vi "Core_Chem_User_Interface_v1.4.vi"() -> ()   [LabVIEW 2014] (continued)
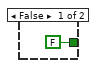
[diagram p11: hidden frame]
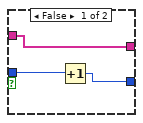
[diagram p16: hidden frame]
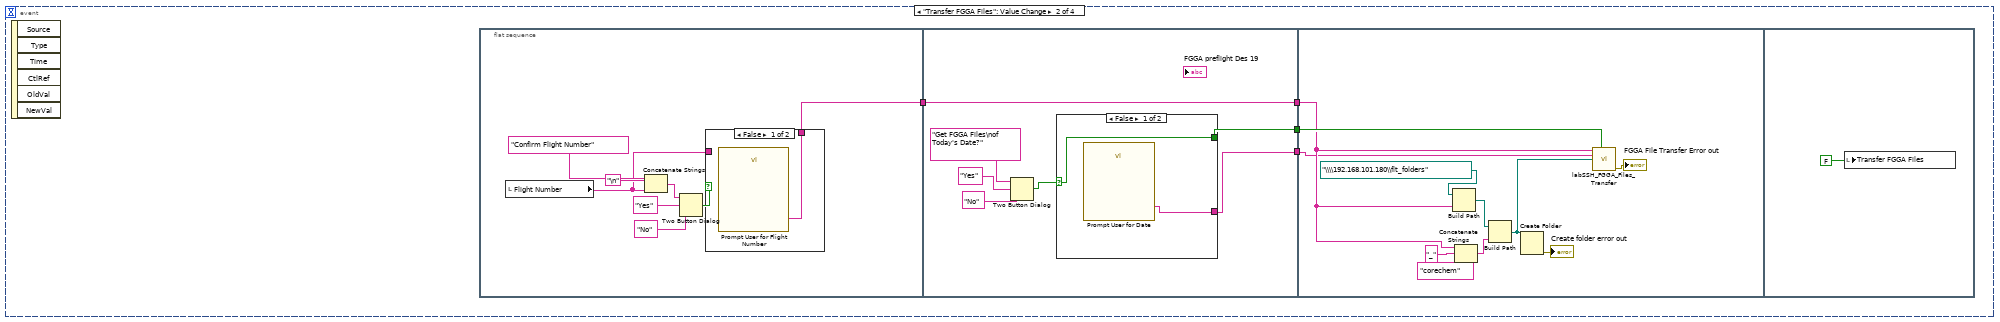
[diagram p18: hidden frame]
            n532 = for {
              N: 60 -> [w1367]
              i -> [w1366]
              n533 = Subtract(x=w1367, y=w1366) -> (x-y=w1365:i32)
              n534 = Decrement(x=w1365) -> (x-1=→"Target Cal\nCal Time Remain (sec)":i32)
              n535 = Wait (ms)(milliseconds to wait=u32 1000) -> ()  [unwired: 1 out]
            }
          }
          frame #5 {
            w1375 = FALSE
            n536 = Cluster To Array(cluster=cluster{"Message 3":string, "Message":string} {"Message 3"="V4", "Message"="V1"}) -> (array=w1373:string[])
            n537 = for {
              tunnel: w1373 -> [w1381] mode=indexing
              tunnel: [w1380] -> w1369
              tunnel: [w1379] -> w1370
              tunnel: w1375 -> [w1378]
              tunnel: w1372 -> [w1377]
              tunnel: w1371 -> [w1376]
              n538 = Bundle(cluster=T4 {"Message"="", "Message Data"=variant} ("Message Cluster"), "Message"=w1381, "Message Data"=w1378) -> (w1383:T4)
              n539 = Enqueue Element(queue=w1377, element=w1383, error in (no error)=w1376) -> (queue out=w1380:refnum<queue>, error out=w1379:errorcluster)  [unwired: 1 in, 1 out]
            }
            n540 = local write "eV4"(w1375) -> ()
            n541 = local write "eV1"(w1375) -> ()
          }
          frame #6 {
            w1385 = 0.0 ("MFC_1\nSLPM Value")
            n542 = local write "MFC_1\nSLPM Value"(w1385) -> ()
            n543 = Bundle(cluster=T4 {"Message"="", "Message Data"=variant} ("Message Cluster"), "Message"="MFC_1", "Message Data"=w1385) -> (w1389:T4)
            n544 = Enqueue Element(queue=w1387, element=w1389, error in (no error)=w1386) -> (error out=w1384:errorcluster)  [unwired: 1 in, 2 out]
          }
          frame #7 {
            n545 = local write "Target Cal"(FALSE ("High Cal")) -> ()
          }
        }
      }
      event "MFC_1\nSLPM Value": Value Change {
        n546 = event-data() -> ()  [unwired: 1 in, 1 out]
        n547 = local read "MFC_1\nSLPM Value"() -> (w1393:dbl)
        n548 = Bundle(cluster=T4 {"Message"="", "Message Data"=variant} ("Message Cluster"), "Message"="MFC_1", "Message Data"=w1393) -> (w1397:T4)
        n549 = Enqueue Element(queue=w1396, element=w1397, error in (no error)=w1395) -> (error out=w1394:errorcluster)  [unwired: 1 in, 2 out]
      }
      event "FGGA UDP Time Offset": Value Change {
        n550 = event-data() -> ("NewVal"=w1400:i32)  [unwired: 1 in, 5 out]
        n551 = Bundle(cluster=T4 {"Message"="", "Message Data"=variant} ("Message Cluster"), "Message"="UDP Time Offset", "Message Data"=w1400) -> (w1404:T4)
        n552 = Enqueue Element(queue=w1403, element=w1404, error in (no error)=w1402) -> (error out=w1401:errorcluster)  [unwired: 1 in, 2 out]
      }
    }
    "FGGA Event Error out" <- w687
  }
  n553 = Create Network Stream Writer Endpoint(6:w53, 7:10 ("writer buffer size"), 9:w55, 10:"//192.168.101.17/command/reader/FGGA" ("reader url"), 11:"/command/writer/FGGA" ("writer name")) -> (0:w52:errorcluster, 3:w51:refnum<k21>)  [unwired: 2 in]
  n554 = node-c288(w11) -> ()  [unwired: 1 out]
  n555 = while {
    tunnel: w2 -> [w1414]
    shift-right: [w1409] -> _
    shift-left: w51 -> [w1411]
    shift-right: [w1407] -> w48
    shift-left: w52 -> [w1413]
    tunnel: w1 -> [w1408]
    stop <- w1407 stop-if-true
    # "FGGA UI Command Sender"
    n556 = Dequeue Element(queue=w1414, error in (no error)=w1408) -> (element=w1410:T4)  [unwired: 1 in, 3 out]
    n557 = Unbundle By Name(w1410) -> ("Message"=w1412:string)
    n558 = case shown="\"UDP Time Offset\"" w1412 {
      tunnel: w1413 -> [w1415 w1419 w1426 w1433 w1440 w1447 w1454 w1461 w1468 w1475 w1482]
      tunnel: w1411 -> [w1416 w1422 w1429 w1436 w1443 w1450 w1457 w1464 w1471 w1478 w1485]
      tunnel: w1410 -> [_ w1421 w1428 w1435 w1442 w1449 w1456 w1463 w1470 w1477 w1484]
      tunnel: [w1415 w1418 w1425 w1432 w1439 w1446 w1453 w1460 w1467 w1474 w1481] -> w1407
      tunnel: [w1416 w1417 w1424 w1431 w1438 w1445 w1452 w1459 w1466 w1473 w1480] -> w1409
      frame "False", Default {
      }
      frame "V1" {
        n559 = shared-variable-write(w1422, w1419, w1421) -> (w1420:refnum<k21>, w1423:errorcluster)  [unwired: 1 in, 1 out]
        n560 = Flush Stream(8:w1423, 11:w1420) -> (0:w1418:errorcluster, 3:w1417:refnum<k21>)  [unwired: 2 in, 1 out]
      }
      frame "MFC_1" {
        n561 = shared-variable-write(w1429, w1426, w1428) -> (w1427:refnum<k21>, w1430:errorcluster)  [unwired: 1 in, 1 out]
        n562 = Flush Stream(8:w1430, 11:w1427) -> (0:w1425:errorcluster, 3:w1424:refnum<k21>)  [unwired: 2 in, 1 out]
      }
      frame "UDP Time Offset" {
        n563 = shared-variable-write(w1436, w1433, w1435) -> (w1434:refnum<k21>, w1437:errorcluster)  [unwired: 1 in, 1 out]
        n564 = Flush Stream(8:w1437, 11:w1434) -> (0:w1432:errorcluster, 3:w1431:refnum<k21>)  [unwired: 2 in, 1 out]
      }
      frame "V2" {
        n565 = shared-variable-write(w1443, w1440, w1442) -> (w1441:refnum<k21>, w1444:errorcluster)  [unwired: 1 in, 1 out]
        n566 = Flush Stream(8:w1444, 11:w1441) -> (0:w1439:errorcluster, 3:w1438:refnum<k21>)  [unwired: 2 in, 1 out]
      }
      frame "V3" {
        n567 = shared-variable-write(w1450, w1447, w1449) -> (w1448:refnum<k21>, w1451:errorcluster)  [unwired: 1 in, 1 out]
        n568 = Flush Stream(8:w1451, 11:w1448) -> (0:w1446:errorcluster, 3:w1445:refnum<k21>)  [unwired: 2 in, 1 out]
      }
      frame "V4" {
        n569 = shared-variable-write(w1457, w1454, w1456) -> (w1455:refnum<k21>, w1458:errorcluster)  [unwired: 1 in, 1 out]
        n570 = Flush Stream(8:w1458, 11:w1455) -> (0:w1453:errorcluster, 3:w1452:refnum<k21>)  [unwired: 2 in, 1 out]
      }
      frame "FGGA_pump" {
        n571 = shared-variable-write(w1464, w1461, w1463) -> (w1462:refnum<k21>, w1465:errorcluster)  [unwired: 1 in, 1 out]
        n572 = Flush Stream(8:w1465, 11:w1462) -> (0:w1460:errorcluster, 3:w1459:refnum<k21>)  [unwired: 2 in, 1 out]
      }
      frame "Flight Number" {
        n573 = shared-variable-write(w1471, w1468, w1470) -> (w1469:refnum<k21>, w1472:errorcluster)  [unwired: 1 in, 1 out]
        n574 = Flush Stream(8:w1472, 11:w1469) -> (0:w1467:errorcluster, 3:w1466:refnum<k21>)  [unwired: 2 in, 1 out]
      }
      frame "FGGA_restart" {
        n575 = shared-variable-write(w1478, w1475, w1477) -> (w1476:refnum<k21>, w1479:errorcluster)  [unwired: 1 in, 1 out]
        n576 = Flush Stream(8:w1479, 11:w1476) -> (0:w1474:errorcluster, 3:w1473:refnum<k21>)  [unwired: 2 in, 1 out]
      }
      frame "Stop File Write" {
        n577 = shared-variable-write(w1485, w1482, w1484) -> (w1483:refnum<k21>, w1486:errorcluster)  [unwired: 1 in, 1 out]
        n578 = Flush Stream(8:w1486, 11:w1483) -> (0:w1481:errorcluster, 3:w1480:refnum<k21>)  [unwired: 2 in, 1 out]
      }
    }
  }
  "FGGA command sender error out" <- w48
  n579 = Obtain Queue(name (unnamed)="SO2_Command", element data type=w37) -> (queue out=w46:refnum<queue>, error out=w39:errorcluster)  [unwired: 3 in, 1 out]
  n580 = while {
    tunnel: w46 -> [w1490]
    tunnel: w39 -> [w1489]
    tunnel: [w1487] -> _
    stop <- FALSE stop-if-true
    # "SO2 UI Event Handler Loop"
    n581 = event shown="[1] \"SO2 Flush\": Value Change" {
      selector: _ -> [_ _ _ _ _ _ _ _ _ _ _ _ _ _ _ _ _ _ _]
      dyn-events: _ -> [_ _ _ _ _ _ _ _ _ _ _ _ _ _ _ _ _ _ _]
      timeout: _ -> [_ _ _ _ _ _ _ _ _ _ _ _ _ _ _ _ _ _ _]
      tunnel: w1490 -> [w1497 w1509 w1558 w1591 w1630 w1699 w1706 w1710 w1717 w1724 w1731 w1738 w1745 w1752 w1759 w1766 w1773 w1781 w1795]
      tunnel: w1489 -> [w1496 w1508 w1557 w1590 w1629 w1698 w1705 w1709 w1716 w1723 w1730 w1737 w1744 w1751 w1758 w1765 w1772 w1780 w1794]
      tunnel: [w1491 w1507 w1556 w1589 _ w1693 w1700 w1708 w1715 w1722 w1729 w1736 w1743 w1750 w1757 w1764 w1771 w1779 w1793] -> w1487
      event "eV9": Value Change {
        n582 = event-data() -> ("NewVal"=w1494:bool)  [unwired: 1 in]
        n583 = Bundle(cluster=T4 {"Message"="", "Message Data"=variant} ("Message Cluster"), "Message"="V9", "Message Data"=w1494) -> (w1492:T4)
        n584 = Enqueue Element(queue=w1497, element=w1492, error in (no error)=w1496) -> (error out=w1491:errorcluster)  [unwired: 1 in, 2 out]
      }
      event "SO2 Flush": Value Change {
        n585 = event-data() -> ()  [unwired: 1 in, 1 out]
        n586 = flat-sequence {
          tunnel: w1509 -> [w1517]
          tunnel: w1508 -> [w1516]
          tunnel: [w1512] -> w1504
          tunnel: [w1510] -> w1502
          tunnel: w1504 -> [w1519]
          tunnel: [w1521] -> w1503
          tunnel: w1502 -> [w1520]
          tunnel: [w1522] -> w1501
          tunnel: w1503 -> [w1528]
          tunnel: [w1528] -> w1506
          tunnel: [w1526] -> w1505
          tunnel: w1501 -> [w1526]
          tunnel: w1506 -> [w1537]
          tunnel: [w1536] -> w1500
          tunnel: w1505 -> [w1538]
          tunnel: [w1534] -> w1498
          tunnel: w1500 -> [w1544]
          tunnel: [w1545] -> w1499
          tunnel: w1498 -> [w1543]
          tunnel: [w1550] -> w1507
          tunnel: w1499 -> [w1550]
          frame #0 {
            w1511 = TRUE ("SO2 Flush")
            n587 = Bundle(cluster=T4 {"Message"="", "Message Data"=variant} ("Message Cluster"), "Message"="V9", "Message Data"=w1511) -> (w1513:T4)
            n588 = local write "eV9"(w1511) -> ()
            n589 = Enqueue Element(queue=w1517, element=w1513, error in (no error)=w1516) -> (queue out=w1510:refnum<queue>, error out=w1512:errorcluster)  [unwired: 1 in, 1 out]
          }
          frame #1 {
            n590 = local read "MFC_2 User Set Value"() -> (w1518:dbl)
            n591 = local write "MFC_2\nSLPM Value"(w1518) -> ()
            n592 = Bundle(cluster=T4 {"Message"="", "Message Data"=variant} ("Message Cluster"), "Message"="MFC_2", "Message Data"=w1518) -> (w1523:T4)
            n593 = Enqueue Element(queue=w1520, element=w1523, error in (no error)=w1519) -> (queue out=w1522:refnum<queue>, error out=w1521:errorcluster)  [unwired: 1 in, 1 out]
          }
          frame #2 {
            n594 = for {
              N: "eV9 Flush User\nset time (sec)" -> [w1532]
              i -> [w1531]
              n595 = Subtract(x=w1532, y=w1531) -> (x-y=w1530:i32)
              n596 = Decrement(x=w1530) -> (x-1=w1529:i32)
              n597 = local write "SO2 Flush\nTime Remain (sec)"(w1529) -> ()
              n598 = Wait (ms)(milliseconds to wait=u32 1000) -> ()  [unwired: 1 out]
            }
          }
          frame #3 {
            w1535 = FALSE
            n599 = Bundle(cluster=T4 {"Message"="", "Message Data"=variant} ("Message Cluster"), "Message"="V9", "Message Data"=w1535) -> (w1539:T4)
            n600 = local write "eV9"(w1535) -> ()
            n601 = Enqueue Element(queue=w1538, element=w1539, error in (no error)=w1537) -> (queue out=w1534:refnum<queue>, error out=w1536:errorcluster)  [unwired: 1 in, 1 out]
          }
          frame #4 {
            w1542 = 0.0 ("MFC_2\nSLPM Value")
            n602 = local write "MFC_2\nSLPM Value"(w1542) -> ()
            n603 = Bundle(cluster=T4 {"Message"="", "Message Data"=variant} ("Message Cluster"), "Message"="MFC_2", "Message Data"=w1542) -> (w1546:T4)
            n604 = Enqueue Element(queue=w1543, element=w1546, error in (no error)=w1544) -> (error out=w1545:errorcluster)  [unwired: 1 in, 2 out]
          }
          frame #5 {
            n605 = local write "SO2 Flush"(FALSE ("SO2 Flush")) -> ()
          }
        }
      }
      event "SO2 Zeroing": Value Change {
        n606 = event-data() -> ()  [unwired: 1 in, 1 out]
        n607 = flat-sequence {
          tunnel: w1558 -> [w1566]
          tunnel: w1557 -> [w1565]
          tunnel: [w1561] -> w1555
          tunnel: [w1559] -> w1551
          tunnel: w1555 -> [w1569]
          tunnel: [w1569] -> w1554
          tunnel: [w1568] -> w1552
          tunnel: w1551 -> [w1568]
          tunnel: w1554 -> [w1577]
          tunnel: [w1576] -> w1553
          tunnel: w1552 -> [w1578]
          tunnel: [w1583] -> w1556
          tunnel: w1553 -> [w1583]
          frame #0 {
            w1560 = TRUE ("SO2 Flush")
            n608 = local write "SO2 eV6"(w1560) -> ()
            n609 = Bundle(cluster=T4 {"Message"="", "Message Data"=variant} ("Message Cluster"), "Message"="V6", "Message Data"=w1560) -> (w1562:T4)
            n610 = Enqueue Element(queue=w1566, element=w1562, error in (no error)=w1565) -> (queue out=w1559:refnum<queue>, error out=w1561:errorcluster)  [unwired: 1 in, 1 out]
          }
          frame #1 {
            # "10 Mins Count down"
            n611 = for {
              N: "eV6 User\nset time (sec)" -> [w1573]
              i -> [w1572]
              n612 = Subtract(x=w1573, y=w1572) -> (x-y=w1571:i32)
              n613 = Decrement(x=w1571) -> (x-1=w1570:i32)
              n614 = local write "SO2 Zeroing\nTime Remain (sec)"(w1570) -> ()
              n615 = Wait (ms)(milliseconds to wait=u32 1000) -> ()  [unwired: 1 out]
            }
          }
          frame #2 {
            w1575 = FALSE
            n616 = Bundle(cluster=T4 {"Message"="", "Message Data"=variant} ("Message Cluster"), "Message"="V6", "Message Data"=w1575) -> (w1579:T4)
            n617 = local write "SO2 eV6"(w1575) -> ()
            n618 = Enqueue Element(queue=w1578, element=w1579, error in (no error)=w1577) -> (error out=w1576:errorcluster)  [unwired: 1 in, 2 out]
          }
          frame #3 {
            n619 = local write "SO2 Zeroing"(FALSE ("SO2 Flush")) -> ()
          }
        }
      }
      event "SO2 Inflight \nZeroing": Value Change {
        n620 = event-data() -> ()  [unwired: 1 in, 1 out]
        n621 = flat-sequence {
          tunnel: w1591 -> [w1599]
          tunnel: w1590 -> [w1598]
          tunnel: [w1594] -> w1588
          tunnel: [w1592] -> w1584
          tunnel: w1588 -> [w1602]
          tunnel: [w1602] -> w1587
          tunnel: [w1601] -> w1585
          tunnel: w1584 -> [w1601]
          tunnel: w1587 -> [w1610]
          tunnel: [w1609] -> w1586
          tunnel: w1585 -> [w1611]
          tunnel: [w1616] -> w1589
          tunnel: w1586 -> [w1616]
          frame #0 {
            w1593 = TRUE ("SO2 Flush")
            n622 = local write "SO2 eV6"(w1593) -> ()
            n623 = Bundle(cluster=T4 {"Message"="", "Message Data"=variant} ("Message Cluster"), "Message"="V6", "Message Data"=w1593) -> (w1595:T4)
            n624 = Enqueue Element(queue=w1599, element=w1595, error in (no error)=w1598) -> (queue out=w1592:refnum<queue>, error out=w1594:errorcluster)  [unwired: 1 in, 1 out]
          }
          frame #1 {
            n625 = for {
              N: "eV6 User set time \n(Inflight) (sec)" -> [w1606]
              i -> [w1605]
              n626 = Subtract(x=w1606, y=w1605) -> (x-y=w1604:i32)
              n627 = Decrement(x=w1604) -> (x-1=w1603:i32)
              n628 = local write "SO2 Zeroing (Inflight)\nTime Remain (sec)"(w1603) -> ()
              n629 = Wait (ms)(milliseconds to wait=u32 1000) -> ()  [unwired: 1 out]
            }
          }
          frame #2 {
            w1608 = FALSE
            n630 = Bundle(cluster=T4 {"Message"="", "Message Data"=variant} ("Message Cluster"), "Message"="V6", "Message Data"=w1608) -> (w1612:T4)
            n631 = local write "SO2 eV6"(w1608) -> ()
            n632 = Enqueue Element(queue=w1611, element=w1612, error in (no error)=w1610) -> (error out=w1609:errorcluster)  [unwired: 1 in, 2 out]
          }
          frame #3 {
            n633 = local write "SO2 Inflight \nZeroing"(FALSE ("SO2 Flush")) -> ()
          }
        }
      }
      event "SO2 CAL": Value Change {
        n634 = event-data() -> ()  [unwired: 1 in, 1 out]
        n635 = flat-sequence {
          tunnel: w1630 -> [w1638]
          tunnel: w1629 -> [w1637]
          tunnel: [w1633] -> w1628
          tunnel: [w1632] -> w1626
          tunnel: w1628 -> [w1642]
          tunnel: [w1641] -> w1627
          tunnel: w1626 -> [w1643]
          tunnel: [w1639] -> w1624
          tunnel: w1627 -> [w1649]
          tunnel: [w1649] -> w1625
          tunnel: w1624 -> [w1647]
          tunnel: [w1647] -> w1623
          tunnel: w1625 -> [w1658]
          tunnel: w1623 -> [w1659]
          tunnel: [w1656] -> w1621
          tunnel: [w1655] -> w1619
          tunnel: [w1664] -> w1622
          tunnel: w1621 -> [w1664]
          tunnel: [w1663] -> w1620
          tunnel: w1619 -> [w1663]
          tunnel: w1622 -> [w1674]
          tunnel: w1620 -> [w1673]
          tunnel: [w1672] -> w1618
          tunnel: [w1671] -> w1617
          tunnel: w1618 -> [w1688]
          tunnel: w1617 -> [w1687]
          frame #0 {
            w1631 = TRUE ("SO2 Flush")
            n636 = Bundle(cluster=T4 {"Message"="", "Message Data"=variant} ("Message Cluster"), "Message"="V9", "Message Data"=w1631) -> (w1634:T4)
            n637 = local write "eV9"(w1631) -> ()
            n638 = Enqueue Element(queue=w1638, element=w1634, error in (no error)=w1637) -> (queue out=w1632:refnum<queue>, error out=w1633:errorcluster)  [unwired: 1 in, 1 out]
          }
          frame #1 {
            n639 = local read "MFC_2 User Set Value"() -> (w1640:dbl)
            n640 = local write "MFC_2\nSLPM Value"(w1640) -> ()
            n641 = Bundle(cluster=T4 {"Message"="", "Message Data"=variant} ("Message Cluster"), "Message"="MFC_2", "Message Data"=w1640) -> (w1644:T4)
            n642 = Enqueue Element(queue=w1643, element=w1644, error in (no error)=w1642) -> (queue out=w1639:refnum<queue>, error out=w1641:errorcluster)  [unwired: 1 in, 1 out]
          }
          frame #2 {
            n643 = for {
              N: "eV9 flush User\nset time (sec)" -> [w1653]
              i -> [w1652]
              n644 = Subtract(x=w1653, y=w1652) -> (x-y=w1651:i32)
              n645 = Decrement(x=w1651) -> (x-1=w1650:i32)
              n646 = local write "SO2 Cal Flush\nTime Remain (sec)"(w1650) -> ()
              n647 = Wait (ms)(milliseconds to wait=u32 1000) -> ()  [unwired: 1 out]
            }
          }
          frame #3 {
            w1657 = TRUE ("SO2 Flush")
            n648 = Bundle(cluster=T4 {"Message"="", "Message Data"=variant} ("Message Cluster"), "Message"="V8", "Message Data"=w1657) -> (w1660:T4)
            n649 = local write "eV8"(w1657) -> ()
            n650 = Enqueue Element(queue=w1659, element=w1660, error in (no error)=w1658) -> (queue out=w1656:refnum<queue>, error out=w1655:errorcluster)  [unwired: 1 in, 1 out]
          }
          frame #4 {
            n651 = for {
              N: "eV8 User\nset time (sec)" -> [w1669]
              i -> [w1668]
              n652 = Subtract(x=w1669, y=w1668) -> (x-y=w1667:i32)
              n653 = Decrement(x=w1667) -> (x-1=w1666:i32)
              n654 = local write "SO2 CAL\nTime Remain (sec)"(w1666) -> ()
              n655 = Wait (ms)(milliseconds to wait=u32 1000) -> ()  [unwired: 1 out]
            }
          }
          frame #5 {
            n656 = Cluster To Array(cluster=cluster{"Message":string, "Message 2":string} {"Message"="V8", "Message 2"="V9"}) -> (array=w1676:string[])
            n657 = for {
              tunnel: w1676 -> [w1683] mode=indexing
              tunnel: FALSE ("SO2 Flush") -> [w1682]
              tunnel: w1674 -> [w1681]
              tunnel: w1673 -> [w1680]
              tunnel: [w1679] -> w1672
              tunnel: [w1678] -> w1671
              n658 = Bundle(cluster=T4 {"Message"="", "Message Data"=variant} ("Message Cluster"), "Message"=w1683, "Message Data"=w1682) -> (w1684:T4)
              n659 = Enqueue Element(queue=w1681, element=w1684, error in (no error)=w1680) -> (queue out=w1679:refnum<queue>, error out=w1678:errorcluster)  [unwired: 1 in, 1 out]
            }
          }
          frame #6 {
            w1686 = 0.0 ("MFC_2\nSLPM Value")
            n660 = local write "MFC_2\nSLPM Value"(w1686) -> ()
            n661 = Bundle(cluster=T4 {"Message"="", "Message Data"=variant} ("Message Cluster"), "Message"="MFC_2", "Message Data"=w1686) -> (w1689:T4)
            n662 = Enqueue Element(queue=w1688, element=w1689, error in (no error)=w1687) -> ()  [unwired: 1 in, 3 out]
          }
          frame #7 {
            w1692 = FALSE ("SO2 Flush")
            n663 = local write "SO2 CAL"(w1692) -> ()
            n664 = local write "eV9"(w1692) -> ()
            n665 = local write "eV8"(w1692) -> ()
          }
        }
      }
      event "MFC_2\nSLPM Value": Value Change {
        n666 = event-data() -> ("NewVal"=w1696:dbl)  [unwired: 1 in]
        n667 = Bundle(cluster=T4 {"Message"="", "Message Data"=variant} ("Message Cluster"), "Message"="MFC_2", "Message Data"=w1696) -> (w1694:T4)
        n668 = Enqueue Element(queue=w1699, element=w1694, error in (no error)=w1698) -> (error out=w1693:errorcluster)  [unwired: 1 in, 2 out]
      }
      event "MFC_3\nSLPM Value": Value Change {
        n669 = event-data() -> ("NewVal"=w1703:dbl)  [unwired: 1 in]
        n670 = Bundle(cluster=T4 {"Message"="", "Message Data"=variant} ("Message Cluster"), "Message"="MFC_3", "Message Data"=w1703) -> (w1701:T4)
        n671 = Enqueue Element(queue=w1706, element=w1701, error in (no error)=w1705) -> (error out=w1700:errorcluster)  [unwired: 1 in, 2 out]
      }
      event "eV8": Value Change {
        n672 = event-data() -> ("NewVal"=w1707:bool)  [unwired: 1 in]
        n673 = Bundle(cluster=T4 {"Message"="", "Message Data"=variant} ("Message Cluster"), "Message"="V8", "Message Data"=w1707) -> (w1711:T4)
        n674 = Enqueue Element(queue=w1710, element=w1711, error in (no error)=w1709) -> (error out=w1708:errorcluster)  [unwired: 1 in, 2 out]
      }
      event "SO2 eV6": Value Change {
        n675 = event-data() -> ("NewVal"=w1714:bool)  [unwired: 1 in]
        n676 = Bundle(cluster=T4 {"Message"="", "Message Data"=variant} ("Message Cluster"), "Message"="V6", "Message Data"=w1714) -> (w1718:T4)
        n677 = Enqueue Element(queue=w1717, element=w1718, error in (no error)=w1716) -> (error out=w1715:errorcluster)  [unwired: 1 in, 2 out]
      }
      event "Simulate Conc": Value Change {
        n678 = event-data() -> ("NewVal"=w1721:bool)  [unwired: 1 in]
        n679 = Bundle(cluster=T4 {"Message"="", "Message Data"=variant} ("Message Cluster"), "Message"="Simulate Conc", "Message Data"=w1721) -> (w1725:T4)
        n680 = Enqueue Element(queue=w1724, element=w1725, error in (no error)=w1723) -> (error out=w1722:errorcluster)  [unwired: 1 in, 2 out]
      }
      event "SO2 UDP Time Offset": Value Change {
        n681 = event-data() -> ("NewVal"=w1728:i32)  [unwired: 1 in]
        n682 = Bundle(cluster=T4 {"Message"="", "Message Data"=variant} ("Message Cluster"), "Message"="UDP Time Offset", "Message Data"=w1728) -> (w1732:T4)
        n683 = Enqueue Element(queue=w1731, element=w1732, error in (no error)=w1730) -> (error out=w1729:errorcluster)  [unwired: 1 in, 2 out]
      }
      event "Simulate STEL Conc": Value Change {
        n684 = event-data() -> ("NewVal"=w1735:dbl)  [unwired: 1 in]
        n685 = Bundle(cluster=T4 {"Message"="", "Message Data"=variant} ("Message Cluster"), "Message"="Simulate STEL Conc", "Message Data"=w1735) -> (w1739:T4)
        n686 = Enqueue Element(queue=w1738, element=w1739, error in (no error)=w1737) -> (error out=w1736:errorcluster)  [unwired: 1 in, 2 out]
      }
      event "Simulate TWA Conc": Value Change {
        n687 = event-data() -> ("NewVal"=w1742:dbl)  [unwired: 1 in]
        n688 = Bundle(cluster=T4 {"Message"="", "Message Data"=variant} ("Message Cluster"), "Message"="Simulate TWA Conc", "Message Data"=w1742) -> (w1746:T4)
        n689 = Enqueue Element(queue=w1745, element=w1746, error in (no error)=w1744) -> (error out=w1743:errorcluster)  [unwired: 1 in, 2 out]
      }
      event "10mins STEL Limit": Value Change {
        n690 = event-data() -> ("NewVal"=w1749:i32)  [unwired: 1 in]
        n691 = Bundle(cluster=T4 {"Message"="", "Message Data"=variant} ("Message Cluster"), "Message"="10mins STEL Limit", "Message Data"=w1749) -> (w1753:T4)
        n692 = Enqueue Element(queue=w1752, element=w1753, error in (no error)=w1751) -> (error out=w1750:errorcluster)  [unwired: 1 in, 2 out]
      }
      event "8hr TWA Limit": Value Change {
        n693 = event-data() -> ("NewVal"=w1756:i32)  [unwired: 1 in]
        n694 = Bundle(cluster=T4 {"Message"="", "Message Data"=variant} ("Message Cluster"), "Message"="8hr TWA Limit", "Message Data"=w1756) -> (w1760:T4)
        n695 = Enqueue Element(queue=w1759, element=w1760, error in (no error)=w1758) -> (error out=w1757:errorcluster)  [unwired: 1 in, 2 out]
      }
      event "SO2 Offset": Value Change {
        n696 = event-data() -> ("NewVal"=w1763:dbl)  [unwired: 1 in]
        n697 = Bundle(cluster=T4 {"Message"="", "Message Data"=variant} ("Message Cluster"), "Message"="Offset", "Message Data"=w1763) -> (w1767:T4)
        n698 = Enqueue Element(queue=w1766, element=w1767, error in (no error)=w1765) -> (error out=w1764:errorcluster)  [unwired: 1 in, 2 out]
      }
      event "SO2 Slope": Value Change {
        n699 = event-data() -> ("NewVal"=w1770:dbl)  [unwired: 1 in]
        n700 = Bundle(cluster=T4 {"Message"="", "Message Data"=variant} ("Message Cluster"), "Message"="Slope", "Message Data"=w1770) -> (w1774:T4)
        n701 = Enqueue Element(queue=w1773, element=w1774, error in (no error)=w1772) -> (error out=w1771:errorcluster)  [unwired: 1 in, 2 out]
      }
      event "Confirm Flight Number": Value Change {
        n702 = event-data() -> ()  [unwired: 1 in, 6 out]
        n703 = flat-sequence {
          tunnel: w1780 -> [w1783]
          tunnel: w1781 -> [w1784]
          tunnel: [w1784] -> w1778
          tunnel: [w1783] -> w1777
          tunnel: [w1786] -> w1779
          tunnel: w1778 -> [w1788]
          tunnel: w1777 -> [w1787]
          frame #0 {
            n704 = local write "cRIO File IO Stop\n(USB Flash Drive Unmount)"(FALSE ("cRIO File IO Stop\n(USB Flash Drive Unmount)")) -> ()
          }
          frame #1 {
            n705 = local read "Flight Number"() -> (w1785:string)
            n706 = Bundle(cluster=T4 {"Message"="", "Message Data"=variant} ("Message Cluster"), "Message"="Flight Number", "Message Data"=w1785) -> (w1789:T4)
            n707 = Enqueue Element(queue=w1788, element=w1789, error in (no error)=w1787) -> (error out=w1786:errorcluster)  [unwired: 1 in, 2 out]
          }
        }
      }
      event "cRIO File IO Stop\n(USB Flash Drive Unmount)": Value Change {
        n708 = event-data() -> ("NewVal"=w1792:bool)  [unwired: 1 in]
        n709 = Bundle(cluster=T4 {"Message"="", "Message Data"=variant} ("Message Cluster"), "Message"="Stop File Write", "Message Data"=w1792) -> (w1796:T4)
        n710 = Enqueue Element(queue=w1795, element=w1796, error in (no error)=w1794) -> (error out=w1793:errorcluster)  [unwired: 1 in, 2 out]
      }
    }
    "SO2 Event error out" <- w1487
  }
  n711 = Create Network Stream Writer Endpoint(6:w43, 7:10 ("writer buffer size"), 9:w37, 10:"//192.168.101.17/command/reader/SO2" ("reader url"), 11:"/command/writer/SO2" ("writer name")) -> (0:w42:errorcluster, 3:w41:refnum<k21>)  [unwired: 2 in]
  n712 = while {
    tunnel: w46 -> [w1806]
    shift-right: [w1801] -> _
    shift-left: w41 -> [w1803]
    shift-right: [w1799] -> w38
    shift-left: w42 -> [w1805]
    tunnel: w39 -> [w1800]
    stop <- w1799 stop-if-true
    # "SO2 UI Command Sender"
    n713 = Dequeue Element(queue=w1806, error in (no error)=w1800) -> (element=w1802:T4)  [unwired: 1 in, 3 out]
    n714 = Unbundle By Name(w1802) -> ("Message"=w1804:string)
    n715 = case shown="\"UDP Time Offset\"" w1804 {
      tunnel: w1805 -> [w1807 w1811 w1818 w1825 w1832 w1839 w1846 w1853 w1860 w1867 w1874 w1881 w1888 w1895 w1902 w1909]
      tunnel: w1803 -> [w1808 w1814 w1821 w1828 w1835 w1842 w1849 w1856 w1863 w1870 w1877 w1884 w1891 w1898 w1905 w1912]
      tunnel: w1802 -> [_ w1813 w1820 w1827 w1834 w1841 w1848 w1855 w1862 w1869 w1876 w1883 w1890 w1897 w1904 w1911]
      tunnel: [w1807 w1810 w1817 w1824 w1831 w1838 w1845 w1852 w1859 w1866 w1873 w1880 w1887 w1894 w1901 w1908] -> w1799
      tunnel: [w1808 w1809 w1816 w1823 w1830 w1837 w1844 w1851 w1858 w1865 w1872 w1879 w1886 w1893 w1900 w1907] -> w1801
      frame "False", Default {
      }
      frame "V9" {
        n716 = shared-variable-write(w1814, w1811, w1813) -> (w1812:refnum<k21>, w1815:errorcluster)  [unwired: 1 in, 1 out]
        n717 = Flush Stream(8:w1815, 11:w1812) -> (0:w1810:errorcluster, 3:w1809:refnum<k21>)  [unwired: 2 in, 1 out]
      }
      frame "MFC_2" {
        n718 = shared-variable-write(w1821, w1818, w1820) -> (w1819:refnum<k21>, w1822:errorcluster)  [unwired: 1 in, 1 out]
        n719 = Flush Stream(8:w1822, 11:w1819) -> (0:w1817:errorcluster, 3:w1816:refnum<k21>)  [unwired: 2 in, 1 out]
      }
      frame "MFC_3" {
        n720 = shared-variable-write(w1828, w1825, w1827) -> (w1826:refnum<k21>, w1829:errorcluster)  [unwired: 1 in, 1 out]
        n721 = Flush Stream(8:w1829, 11:w1826) -> (0:w1824:errorcluster, 3:w1823:refnum<k21>)  [unwired: 2 in, 1 out]
      }
      frame "V6" {
        n722 = shared-variable-write(w1835, w1832, w1834) -> (w1833:refnum<k21>, w1836:errorcluster)  [unwired: 1 in, 1 out]
        n723 = Flush Stream(8:w1836, 11:w1833) -> (0:w1831:errorcluster, 3:w1830:refnum<k21>)  [unwired: 2 in, 1 out]
      }
      frame "Simulate Conc" {
        n724 = shared-variable-write(w1842, w1839, w1841) -> (w1840:refnum<k21>, w1843:errorcluster)  [unwired: 1 in, 1 out]
        n725 = Flush Stream(8:w1843, 11:w1840) -> (0:w1838:errorcluster, 3:w1837:refnum<k21>)  [unwired: 2 in, 1 out]
      }
      frame "Simulate STEL Conc" {
        n726 = shared-variable-write(w1849, w1846, w1848) -> (w1847:refnum<k21>, w1850:errorcluster)  [unwired: 1 in, 1 out]
        n727 = Flush Stream(8:w1850, 11:w1847) -> (0:w1845:errorcluster, 3:w1844:refnum<k21>)  [unwired: 2 in, 1 out]
      }
      frame "Simulate TWA Conc" {
        n728 = shared-variable-write(w1856, w1853, w1855) -> (w1854:refnum<k21>, w1857:errorcluster)  [unwired: 1 in, 1 out]
        n729 = Flush Stream(8:w1857, 11:w1854) -> (0:w1852:errorcluster, 3:w1851:refnum<k21>)  [unwired: 2 in, 1 out]
      }
      frame "10mins STEL Limit" {
        n730 = shared-variable-write(w1863, w1860, w1862) -> (w1861:refnum<k21>, w1864:errorcluster)  [unwired: 1 in, 1 out]
        n731 = Flush Stream(8:w1864, 11:w1861) -> (0:w1859:errorcluster, 3:w1858:refnum<k21>)  [unwired: 2 in, 1 out]
      }
      frame "8hr TWA Limit" {
        n732 = shared-variable-write(w1870, w1867, w1869) -> (w1868:refnum<k21>, w1871:errorcluster)  [unwired: 1 in, 1 out]
        n733 = Flush Stream(8:w1871, 11:w1868) -> (0:w1866:errorcluster, 3:w1865:refnum<k21>)  [unwired: 2 in, 1 out]
      }
      frame "Offset" {
        n734 = shared-variable-write(w1877, w1874, w1876) -> (w1875:refnum<k21>, w1878:errorcluster)  [unwired: 1 in, 1 out]
        n735 = Flush Stream(8:w1878, 11:w1875) -> (0:w1873:errorcluster, 3:w1872:refnum<k21>)  [unwired: 2 in, 1 out]
      }
      frame "Slope" {
        n736 = shared-variable-write(w1884, w1881, w1883) -> (w1882:refnum<k21>, w1885:errorcluster)  [unwired: 1 in, 1 out]
        n737 = Flush Stream(8:w1885, 11:w1882) -> (0:w1880:errorcluster, 3:w1879:refnum<k21>)  [unwired: 2 in, 1 out]
      }
      frame "Flight Number" {
        n738 = shared-variable-write(w1891, w1888, w1890) -> (w1889:refnum<k21>, w1892:errorcluster)  [unwired: 1 in, 1 out]
        n739 = Flush Stream(8:w1892, 11:w1889) -> (0:w1887:errorcluster, 3:w1886:refnum<k21>)  [unwired: 2 in, 1 out]
      }
      frame "Stop File Write" {
        n740 = shared-variable-write(w1898, w1895, w1897) -> (w1896:refnum<k21>, w1899:errorcluster)  [unwired: 1 in, 1 out]
        n741 = Flush Stream(8:w1899, 11:w1896) -> (0:w1894:errorcluster, 3:w1893:refnum<k21>)  [unwired: 2 in, 1 out]
      }
      frame "UDP Time Offset" {
        n742 = shared-variable-write(w1905, w1902, w1904) -> (w1903:refnum<k21>, w1906:errorcluster)  [unwired: 1 in, 1 out]
        n743 = Flush Stream(8:w1906, 11:w1903) -> (0:w1901:errorcluster, 3:w1900:refnum<k21>)  [unwired: 2 in, 1 out]
      }
      frame "V8" {
        n744 = shared-variable-write(w1912, w1909, w1911) -> (w1910:refnum<k21>, w1913:errorcluster)  [unwired: 1 in, 1 out]
        n745 = Flush Stream(8:w1913, 11:w1910) -> (0:w1908:errorcluster, 3:w1907:refnum<k21>)  [unwired: 2 in, 1 out]
      }
    }
  }
  "SO2 command sender \nerror out" <- w38
  n746 = Obtain Queue(name (unnamed)="TEi43c_Command", element data type=w26) -> (queue out=w35:refnum<queue>, error out=w28:errorcluster)  [unwired: 3 in, 1 out]
  n747 = Create Network Stream Writer Endpoint(6:w32, 7:10 ("writer buffer size"), 9:w26, 10:"//192.168.101.17/command/reader/TEi43c" ("reader url"), 11:"/command/writer/TEi43c" ("writer name")) -> (0:w31:errorcluster, 3:w30:refnum<k21>)  [unwired: 2 in]
  n748 = while {
    tunnel: w35 -> [w1917]
    tunnel: w28 -> [w1916]
    tunnel: [w1914] -> _
    stop <- FALSE stop-if-true
    # "TEi43c Ozone UI Event Handler Loop"
    n749 = event shown="[4] \"Confirm Flight Number\": Value Change" {
      selector: _ -> [_ _ _ _ _]
      dyn-events: _ -> [_ _ _ _ _]
      timeout: _ -> [_ _ _ _ _]
      tunnel: w1917 -> [w1925 w1953 w1961 w1968 w1976]
      tunnel: w1916 -> [w1924 w1952 w1960 w1967 w1975]
      tunnel: [w1923 w1951 w1959 w1966 w1974] -> w1914
      event "Ozone Zeroing": Value Change {
        n750 = event-data() -> ()  [unwired: 1 in, 6 out]
        n751 = flat-sequence {
          tunnel: w1925 -> [w1930]
          tunnel: w1924 -> [w1929]
          tunnel: [w1928] -> w1922
          tunnel: [w1926] -> w1918
          tunnel: w1922 -> [w1936]
          tunnel: [w1936] -> w1921
          tunnel: [w1934] -> w1919
          tunnel: w1918 -> [w1934]
          tunnel: w1921 -> [w1944]
          tunnel: [w1943] -> w1920
          tunnel: w1919 -> [w1945]
          tunnel: [w1950] -> w1923
          tunnel: w1920 -> [w1950]
          frame #0 {
            w1927 = TRUE
            n752 = local write "Ozone eV6"(w1927) -> ()
            n753 = Bundle(cluster=T4 {"Message"="", "Message Data"=variant} ("Message Cluster"), "Message"="V6", "Message Data"=w1927) -> (w1931:T4)
            n754 = Enqueue Element(queue=w1930, element=w1931, error in (no error)=w1929) -> (queue out=w1926:refnum<queue>, error out=w1928:errorcluster)  [unwired: 1 in, 1 out]
          }
          frame #1 {
            # "10 Mins Count down"
            n755 = for {
              N: 600 -> [w1940]
              i -> [w1939]
              n756 = Subtract(x=w1940, y=w1939) -> (x-y=w1938:i32)
              n757 = Decrement(x=w1938) -> (x-1=→"Ozone Zeroing\nTime Remain (sec)":i32)
              n758 = Wait (ms)(milliseconds to wait=u32 1000) -> ()  [unwired: 1 out]
            }
          }
          frame #2 {
            w1942 = FALSE
            n759 = local write "Ozone eV6"(w1942) -> ()
            n760 = Bundle(cluster=T4 {"Message"="", "Message Data"=variant} ("Message Cluster"), "Message"="V6", "Message Data"=w1942) -> (w1946:T4)
            n761 = Enqueue Element(queue=w1945, element=w1946, error in (no error)=w1944) -> (error out=w1943:errorcluster)  [unwired: 1 in, 2 out]
          }
          frame #3 {
            n762 = local write "Ozone Zeroing"(FALSE ("Ozone Zeroing")) -> ()
          }
        }
      }
      event "Ozone eV6": Value Change {
        n763 = event-data() -> ("NewVal"=w1954:bool)  [unwired: 1 in]
        n764 = Bundle(cluster=T4 {"Message"="", "Message Data"=variant} ("Message Cluster"), "Message"="V6", "Message Data"=w1954) -> (w1955:T4)
        n765 = Enqueue Element(queue=w1953, element=w1955, error in (no error)=w1952) -> (error out=w1951:errorcluster)  [unwired: 1 in, 2 out]
      }
      event "cRIO File IO Stop\n(USB Flash Drive Unmount)": Value Change {
        n766 = event-data() -> ("NewVal"=w1958:bool)  [unwired: 1 in]
        n767 = Bundle(cluster=T4 {"Message"="", "Message Data"=variant} ("Message Cluster"), "Message"="Stop File Write", "Message Data"=w1958) -> (w1962:T4)
        n768 = Enqueue Element(queue=w1961, element=w1962, error in (no error)=w1960) -> (error out=w1959:errorcluster)  [unwired: 1 in, 2 out]
      }
      event "Ozone UDP Time Offset": Value Change {
        n769 = event-data() -> ("NewVal"=w1965:i32)  [unwired: 1 in]
        n770 = Bundle(cluster=T4 {"Message"="", "Message Data"=variant} ("Message Cluster"), "Message"="UDP Time Offset", "Message Data"=w1965) -> (w1969:T4)
        n771 = Enqueue Element(queue=w1968, element=w1969, error in (no error)=w1967) -> (error out=w1966:errorcluster)  [unwired: 1 in, 2 out]
      }
      event "Confirm Flight Number": Value Change {
        n772 = event-data() -> ()  [unwired: 1 in, 5 out]
        n773 = flat-sequence {
          tunnel: w1975 -> [w1978]
          tunnel: w1976 -> [w1979]
          tunnel: [w1979] -> w1973
          tunnel: [w1978] -> w1972
          tunnel: [w1981] -> w1974
          tunnel: w1973 -> [w1983]
          tunnel: w1972 -> [w1982]
          frame #0 {
            n774 = local write "cRIO File IO Stop\n(USB Flash Drive Unmount)"(FALSE ("cRIO File IO Stop\n(USB Flash Drive Unmount)")) -> ()
          }
          frame #1 {
            n775 = local read "Flight Number"() -> (w1980:string)
            n776 = Bundle(cluster=T4 {"Message"="", "Message Data"=variant} ("Message Cluster"), "Message"="Flight Number", "Message Data"=w1980) -> (w1984:T4)
            n777 = Enqueue Element(queue=w1983, element=w1984, error in (no error)=w1982) -> (error out=w1981:errorcluster)  [unwired: 1 in, 2 out]
          }
        }
      }
    }
    "Ozone Event error out" <- w1914
  }
  n778 = while {
    tunnel: w35 -> [w1994]
    shift-right: [w1989] -> _
    shift-left: w30 -> [w1991]
    shift-right: [w1987] -> w27
    shift-left: w31 -> [w1993]
    tunnel: w28 -> [w1988]
    stop <- w1987 stop-if-true
    # "TEi43c Ozone UI Command Sender"
    n779 = Dequeue Element(queue=w1994, error in (no error)=w1988) -> (element=w1990:T4)  [unwired: 1 in, 3 out]
    n780 = Unbundle By Name(w1990) -> ("Message"=w1992:string)
    n781 = case shown="\"UDP Time Offset\"" w1992 {
      tunnel: w1993 -> [w1995 w1999 w2006 w2013 w2020]
      tunnel: w1991 -> [w1996 w2002 w2009 w2016 w2023]
      tunnel: w1990 -> [_ w2001 w2008 w2015 w2022]
      tunnel: [w1995 w1998 w2005 w2012 w2019] -> w1987
      tunnel: [w1996 w1997 w2004 w2011 w2018] -> w1989
      frame "False", Default {
      }
      frame "V6" {
        n782 = shared-variable-write(w2002, w1999, w2001) -> (w2000:refnum<k21>, w2003:errorcluster)  [unwired: 1 in, 1 out]
        n783 = Flush Stream(8:w2003, 11:w2000) -> (0:w1998:errorcluster, 3:w1997:refnum<k21>)  [unwired: 2 in, 1 out]
      }
      frame "Stop File Write" {
        n784 = shared-variable-write(w2009, w2006, w2008) -> (w2007:refnum<k21>, w2010:errorcluster)  [unwired: 1 in, 1 out]
        n785 = Flush Stream(8:w2010, 11:w2007) -> (0:w2005:errorcluster, 3:w2004:refnum<k21>)  [unwired: 2 in, 1 out]
      }
      frame "Flight Number" {
        n786 = shared-variable-write(w2016, w2013, w2015) -> (w2014:refnum<k21>, w2017:errorcluster)  [unwired: 1 in, 1 out]
        n787 = Flush Stream(8:w2017, 11:w2014) -> (0:w2012:errorcluster, 3:w2011:refnum<k21>)  [unwired: 2 in, 1 out]
      }
      frame "UDP Time Offset" {
        n788 = shared-variable-write(w2023, w2020, w2022) -> (w2021:refnum<k21>, w2024:errorcluster)  [unwired: 1 in, 1 out]
        n789 = Flush Stream(8:w2024, 11:w2021) -> (0:w2019:errorcluster, 3:w2018:refnum<k21>)  [unwired: 2 in, 1 out]
      }
    }
  }
  "Ozone command sender error out" <- w27
  n790 = Obtain Queue(name (unnamed)="2BOzone_Command", element data type=w14) -> (queue out=w23:refnum<queue>, error out=w16:errorcluster)  [unwired: 3 in, 1 out]
  n791 = Create Network Stream Writer Endpoint(6:w20, 7:10 ("writer buffer size"), 9:w14, 10:"//192.168.101.17/command/reader/2BOzone" ("reader url"), 11:"/command/writer/2BOzone" ("writer name")) -> (0:w19:errorcluster, 3:w18:refnum<k21>)  [unwired: 2 in]
  n792 = while {
    tunnel: w23 -> [w2028]
    tunnel: w16 -> [w2027]
    tunnel: [w2025] -> _
    stop <- FALSE stop-if-true
    # "2BOzone UI Event Handler Loop"
    n793 = event shown="[7] \"Confirm Flight Number\": Value Change" {
      selector: _ -> [_ _ _ _ _ _ _ _]
      dyn-events: _ -> [_ _ _ _ _ _ _ _]
      timeout: _ -> [_ _ _ _ _ _ _ _]
      tunnel: w2028 -> [w2032 w2039 w2046 w2053 w2060 w2067 w2074 w2082]
      tunnel: w2027 -> [w2031 w2038 w2045 w2052 w2059 w2066 w2073 w2081]
      tunnel: [w2030 w2037 w2044 w2051 w2058 w2065 w2072 w2080] -> w2025
      event "Ambient = OFF\nCabin = ON": Value Change {
        n794 = event-data() -> ("NewVal"=w2029:bool)  [unwired: 1 in]
        n795 = Bundle(cluster=T4 {"Message"="", "Message Data"=variant} ("Message Cluster"), "Message"="Ambient/Cabin", "Message Data"=w2029) -> (w2033:T4)
        n796 = Enqueue Element(queue=w2032, element=w2033, error in (no error)=w2031) -> (error out=w2030:errorcluster)  [unwired: 1 in, 2 out]
      }
      event "Simulate 2B Conc": Value Change {
        n797 = event-data() -> ("NewVal"=w2036:bool)  [unwired: 1 in]
        n798 = Bundle(cluster=T4 {"Message"="", "Message Data"=variant} ("Message Cluster"), "Message"="Simulate_conc", "Message Data"=w2036) -> (w2040:T4)
        n799 = Enqueue Element(queue=w2039, element=w2040, error in (no error)=w2038) -> (error out=w2037:errorcluster)  [unwired: 1 in, 2 out]
      }
      event "Simulate Inst Conc": Value Change {
        n800 = event-data() -> ("NewVal"=w2043:i32)  [unwired: 1 in]
        n801 = Bundle(cluster=T4 {"Message"="", "Message Data"=variant} ("Message Cluster"), "Message"="Simulate_inst_conc", "Message Data"=w2043) -> (w2047:T4)
        n802 = Enqueue Element(queue=w2046, element=w2047, error in (no error)=w2045) -> (error out=w2044:errorcluster)  [unwired: 1 in, 2 out]
      }
      event "Inst_alm_thresh": Value Change {
        n803 = event-data() -> ("NewVal"=w2050:i32)  [unwired: 1 in]
        n804 = Bundle(cluster=T4 {"Message"="", "Message Data"=variant} ("Message Cluster"), "Message"="Inst_alm_thresh", "Message Data"=w2050) -> (w2054:T4)
        n805 = Enqueue Element(queue=w2053, element=w2054, error in (no error)=w2052) -> (error out=w2051:errorcluster)  [unwired: 1 in, 2 out]
      }
      event "3hr_alm_thresh": Value Change {
        n806 = event-data() -> ("NewVal"=w2057:i32)  [unwired: 1 in]
        n807 = Bundle(cluster=T4 {"Message"="", "Message Data"=variant} ("Message Cluster"), "Message"="3hr_alm_thresh", "Message Data"=w2057) -> (w2061:T4)
        n808 = Enqueue Element(queue=w2060, element=w2061, error in (no error)=w2059) -> (error out=w2058:errorcluster)  [unwired: 1 in, 2 out]
      }
      event "Simulate 3hr Average Conc": Value Change {
        n809 = event-data() -> ("NewVal"=w2064:dbl)  [unwired: 1 in]
        n810 = Bundle(cluster=T4 {"Message"="", "Message Data"=variant} ("Message Cluster"), "Message"="Simulate_3hr_av_conc", "Message Data"=w2064) -> (w2068:T4)
        n811 = Enqueue Element(queue=w2067, element=w2068, error in (no error)=w2066) -> (error out=w2065:errorcluster)  [unwired: 1 in, 2 out]
      }
      event "cRIO File IO Stop\n(USB Flash Drive Unmount)": Value Change {
        n812 = event-data() -> ("NewVal"=w2071:bool)  [unwired: 1 in]
        n813 = Bundle(cluster=T4 {"Message"="", "Message Data"=variant} ("Message Cluster"), "Message"="Stop File Write", "Message Data"=w2071) -> (w2075:T4)
        n814 = Enqueue Element(queue=w2074, element=w2075, error in (no error)=w2073) -> (error out=w2072:errorcluster)  [unwired: 1 in, 2 out]
      }
      event "Confirm Flight Number": Value Change {
        n815 = event-data() -> ()  [unwired: 1 in, 5 out]
        n816 = flat-sequence {
          tunnel: w2081 -> [w2084]
          tunnel: w2082 -> [w2085]
          tunnel: [w2085] -> w2079
          tunnel: [w2084] -> w2078
          tunnel: [w2087] -> w2080
          tunnel: w2079 -> [w2089]
          tunnel: w2078 -> [w2088]
          frame #0 {
            n817 = local write "cRIO File IO Stop\n(USB Flash Drive Unmount)"(FALSE ("cRIO File IO Stop\n(USB Flash Drive Unmount)")) -> ()
          }
          frame #1 {
            n818 = local read "Flight Number"() -> (w2086:string)
            n819 = Bundle(cluster=T4 {"Message"="", "Message Data"=variant} ("Message Cluster"), "Message"="Flight Number", "Message Data"=w2086) -> (w2090:T4)
            n820 = Enqueue Element(queue=w2089, element=w2090, error in (no error)=w2088) -> (error out=w2087:errorcluster)  [unwired: 1 in, 2 out]
          }
        }
      }
    }
    "2BOzone Event error out" <- w2025
  }
  n821 = while {
    tunnel: w23 -> [w2100]
    shift-right: [w2095] -> _
    shift-left: w18 -> [w2097]
    shift-right: [w2093] -> w15
    shift-left: w19 -> [w2099]
    tunnel: w16 -> [w2094]
    stop <- w2093 stop-if-true
    # "2BOzone UI Command Sender"
    n822 = Dequeue Element(queue=w2100, error in (no error)=w2094) -> (element=w2096:T4)  [unwired: 1 in, 3 out]
    n823 = Unbundle By Name(w2096) -> ("Message"=w2098:string)
    n824 = case shown="\"3hr_alm_thresh\"" w2098 {
      tunnel: w2099 -> [w2101 w2105 w2112 w2119 w2126 w2133 w2140 w2147 w2154]
      tunnel: w2097 -> [w2102 w2108 w2115 w2122 w2129 w2136 w2143 w2150 w2157]
      tunnel: w2096 -> [_ w2107 w2114 w2121 w2128 w2135 w2142 w2149 w2156]
      tunnel: [w2101 w2104 w2111 w2118 w2125 w2132 w2139 w2146 w2153] -> w2093
      tunnel: [w2102 w2103 w2110 w2117 w2124 w2131 w2138 w2145 w2152] -> w2095
      frame "False", Default {
      }
      frame "Ambient/Cabin" {
        n825 = shared-variable-write(w2108, w2105, w2107) -> (w2106:refnum<k21>, w2109:errorcluster)  [unwired: 1 in, 1 out]
        n826 = Flush Stream(8:w2109, 11:w2106) -> (0:w2104:errorcluster, 3:w2103:refnum<k21>)  [unwired: 2 in, 1 out]
      }
      frame "Simulate_conc" {
        n827 = shared-variable-write(w2115, w2112, w2114) -> (w2113:refnum<k21>, w2116:errorcluster)  [unwired: 1 in, 1 out]
        n828 = Flush Stream(8:w2116, 11:w2113) -> (0:w2111:errorcluster, 3:w2110:refnum<k21>)  [unwired: 2 in, 1 out]
      }
      frame "Simulate_inst_conc" {
        n829 = shared-variable-write(w2122, w2119, w2121) -> (w2120:refnum<k21>, w2123:errorcluster)  [unwired: 1 in, 1 out]
        n830 = Flush Stream(8:w2123, 11:w2120) -> (0:w2118:errorcluster, 3:w2117:refnum<k21>)  [unwired: 2 in, 1 out]
      }
      frame "Inst_alm_thresh" {
        n831 = shared-variable-write(w2129, w2126, w2128) -> (w2127:refnum<k21>, w2130:errorcluster)  [unwired: 1 in, 1 out]
        n832 = Flush Stream(8:w2130, 11:w2127) -> (0:w2125:errorcluster, 3:w2124:refnum<k21>)  [unwired: 2 in, 1 out]
      }
      frame "3hr_alm_thresh" {
        n833 = shared-variable-write(w2136, w2133, w2135) -> (w2134:refnum<k21>, w2137:errorcluster)  [unwired: 1 in, 1 out]
        n834 = Flush Stream(8:w2137, 11:w2134) -> (0:w2132:errorcluster, 3:w2131:refnum<k21>)  [unwired: 2 in, 1 out]
      }
      frame "Simulate_3hr_av_conc" {
        n835 = shared-variable-write(w2143, w2140, w2142) -> (w2141:refnum<k21>, w2144:errorcluster)  [unwired: 1 in, 1 out]
        n836 = Flush Stream(8:w2144, 11:w2141) -> (0:w2139:errorcluster, 3:w2138:refnum<k21>)  [unwired: 2 in, 1 out]
      }
      frame "Stop File Write" {
        n837 = shared-variable-write(w2150, w2147, w2149) -> (w2148:refnum<k21>, w2151:errorcluster)  [unwired: 1 in, 1 out]
        n838 = Flush Stream(8:w2151, 11:w2148) -> (0:w2146:errorcluster, 3:w2145:refnum<k21>)  [unwired: 2 in, 1 out]
      }
      frame "Flight Number" {
        n839 = shared-variable-write(w2157, w2154, w2156) -> (w2155:refnum<k21>, w2158:errorcluster)  [unwired: 1 in, 1 out]
        n840 = Flush Stream(8:w2158, 11:w2155) -> (0:w2153:errorcluster, 3:w2152:refnum<k21>)  [unwired: 2 in, 1 out]
      }
    }
  }
  "2BOzone command sender error out" <- w15
